vi "SimulatedImageProcessing.vi"() -> ()   [LabVIEW 2011]
uses:
  <vilib>/vision/Image Controls.llb/IMAQ Image.ctl
panel:
  in  "threshold":cluster{"Lower value":sgl, "Upper value":sgl}={"Lower value"=0.0, "Upper value"=100.0}
  out "# of Particles found":i32=1
  in  "remove particle size":i32=5
  in  "Operation":u16(ring)=3 items=["AutoM", "Close", "Dilate", "Erode", "Gradient", "Gradient out", "Gradient in", "Hit miss", "Open", "PClose", "POpen", "Thick", "Thin"]
  in  "Interpolation Type":u32(ring)=1 items=["Zero Order", "Bi-Linear", "Quadratic", "Cubic Spline"]
  in  "downsampling":u32=10
  out "Image Out 3":T1(plugin-control)
  out "Image Out 2":T1(plugin-control)
  out "Frame Rate":dbl=23.346303501945524
  out "Image Out":T1(plugin-control)
  in  "Stop (F)":bool
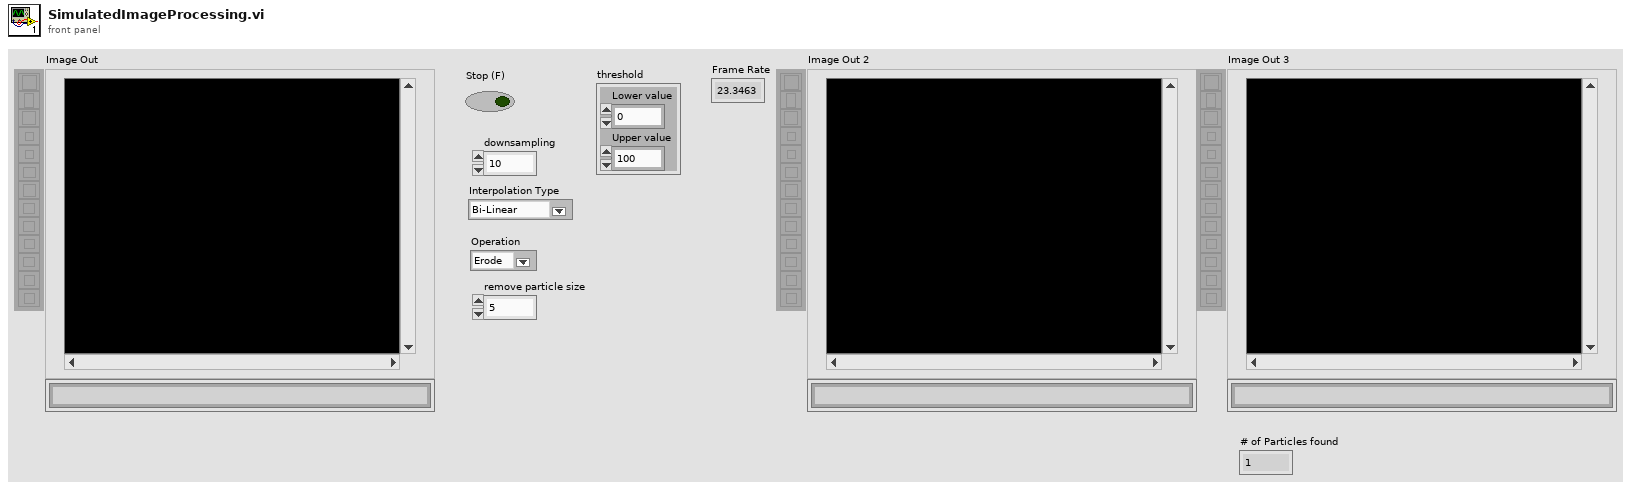
[diagram p1: front panel]
types:
  T1 = typedef "IMAQ Image.ctl" = refnum<image>
  T2 = cluster{"Channel":i32, "Range":cluster{"Lower value":sgl, "Upper value":sgl}, "downsampling":u32, "Operation":u16, "Interpolation Type":u32, "remove particle size":i32, "Single channel":T1, "Thresholded":T1, "raw image":T1}
  T3 = cluster{"Buffer Number":u32, "Frame Rate":dbl, "# of Particles found":i32, "Image":T1, "Single channel":T1, "thresholded":T1, "status":bool}
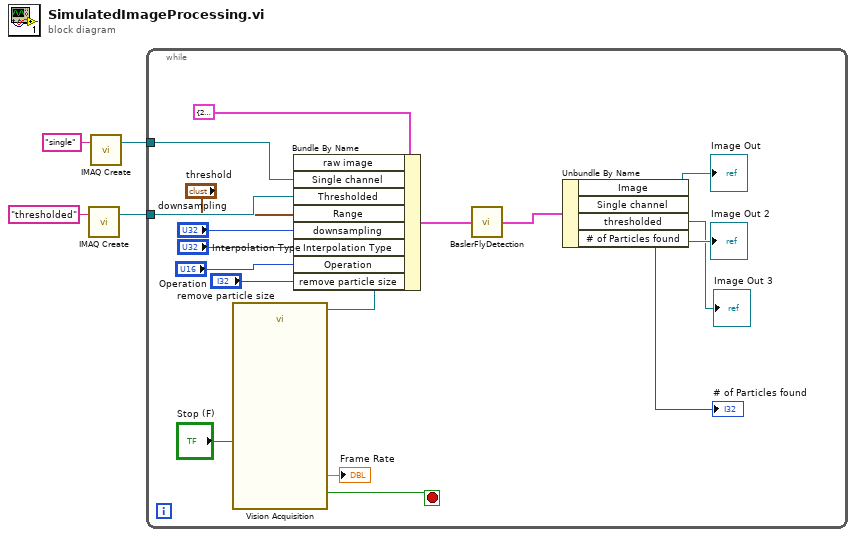
[diagram p0: block diagram]
diagram:
  n1 = call "IMAQ Create"("Image Name"="thresholded") -> ("New Image"=w1:T1)  [unwired: 3 in, 2 out]
  n2 = call "IMAQ Create"("Image Name"="single") -> ("New Image"=w2:T1)  [unwired: 3 in, 2 out]
  n3 = while {
    tunnel: w2 -> [w16]
    tunnel: w1 -> [w15]
    stop <- w21 stop-if-true
    n4 = call "Vision Acquisition"("Stop (F)"="Stop (F)") -> ("Image Out"=w17:T1, "Frame Rate"=→"Frame Rate":dbl, "Stopped"=w21:bool)  [unwired: 22 in, 2 out]
    n5 = Bundle By Name(cluster=T2 {"Channel"=2, "Range"={"Lower value"=0.0, "Upper value"=100.0}, "downsampling"=4, "Operation"=0, "Interpolation Type"=1, "remove particle size"=1, "Single channel"="single", "Thresholded"="thresholded", "raw image"="Vision Acq Image 47498962Untitled 1:Instance:0<Not A Path>"} ("image processing controls"), "raw image"=w17, "Single channel"=w16, "Thresholded"=w15, "Range"="threshold", "downsampling"="downsampling", "Interpolation Type"="Interpolation Type", "Operation"="Operation", "remove particle size"="remove particle size") -> (w18:T2)
    n6 = call "BaslerFlyDetection.vi"("image processing controls"=w18) -> ("image processing indicators"=w10:T3)
    n7 = Unbundle By Name(w10) -> ("Image"=→"Image Out":T1, "Single channel"=→"Image Out 2":T1, "thresholded"=→"Image Out 3":T1, "# of Particles found"=→"# of Particles found":i32)
  }
